vi "Dresden R2R Sputter 03.02.2018 IY24.vi"() -> ()   [LabVIEW 2009] (continued)
              }
              frame #1 {
                n8490 = call "Elapsed Time120"("Reset"=w13371) -> ("Elapsed Time (s)"=w13370:dbl)  [unwired: 11 in, 7 out]
                n8491 = Greater?(x=w13370, y=5.0) -> (0:w13368:bool)
              }
            }
            n8492 = local write "ch3_cc_fail_top"(w13330) -> ()
            n8493 = local write "Ch3_Ch_cc_fail"(w13330) -> ()
          }
        }
        n8494 = case shown="False" w13260 {
          frame #0 {
            n8495 = local read "Ch3_Trns_gv_bp2_do"() -> (w13266:bool)
            n8496 = local read "Ch3_Trns_gv_bp2_di"() -> (w13267:bool)
            n8497 = Exclusive Or(1:w13266, 2:w13267) -> (0:w13265:bool)
            n8498 = feedback #272() -> (w13264:bool)  [unwired: 1 in]
            n8499 = case shown="True" w13265 {
              tunnel: [TRUE FALSE] -> w13263
              tunnel: w13264 -> [_ w13273]
              tunnel: [FALSE w13270] -> w13262
              frame #0 {
              }
              frame #1 {
                n8500 = call "Elapsed Time156"("Reset"=w13273) -> ("Elapsed Time (s)"=w13272:dbl)  [unwired: 11 in, 7 out]
                n8501 = Greater?(x=w13272, y=5.0) -> (0:w13270:bool)
              }
            }
            n8502 = local write "Ch3_trns_gv_bp2_fail_front"(w13262) -> ()
            n8503 = local write "Ch3_Trns_gv_bp2_fail"(w13262) -> ()
            n8504 = local write "ch3_trns_gv_bp2_on_top"(w13262) -> ()
          }
          frame #1 {
            w13275 = TRUE ("Ch_bv_fail(ch3)L")
            n8505 = local write "Ch3_Trns_gv_bp2_fail"(w13275) -> ()
            n8506 = local write "Ch3_trns_gv_bp2_fail_front"(w13275) -> ()
            n8507 = local write "ch3_trns_gv_bp2_on_top"(w13275) -> ()
          }
        }
        n8508 = case shown="False" w13259 {
          frame #0 {
          }
          frame #1 {
          }
        }
        n8509 = case shown="False" w13261 {
          frame #0 {
            w13276 = TRUE ("Mp_fail(ch3)")
            n8510 = local write "Trns_gv_3_4_fail"(w13276) -> ()
            n8511 = local write "ch3_sov_Ar_fail_top"(w13276) -> ()
            n8512 = local write "gv top failed ch4_3"(w13276) -> ()
            n8513 = local write "gv front failed ch4_3"(w13276) -> ()
            n8514 = local write "gv top failed_ch3_4"(w13276) -> ()
            n8515 = local write "gv front failed_ch3_4"(w13276) -> ()
            n8516 = local write "Ch3_Trns_gv_bp_fail"(w13276) -> ()
            n8517 = local write "ch3_trns_gv_bp_on_top"(w13276) -> ()
            n8518 = local write "Ch3_trns_gv_bp_fail_front"(w13276) -> ()
            n8519 = local write "chamber 3 top piston failed"(w13276) -> ()
          }
          frame #1 {
            n8520 = local read "Ch3_Sov_Ar_do"() -> (w13296:bool)
            n8521 = local read "Ch3_Sov_Ar_di"() -> (w13297:bool)
            n8522 = Exclusive Or(1:w13296, 2:w13297) -> (0:w13298:bool)
            n8523 = feedback #273() -> (w13299:bool)  [unwired: 1 in]
            n8524 = case shown="True" w13298 {
              tunnel: [TRUE FALSE] -> w13300
              tunnel: w13299 -> [_ w13327]
              tunnel: [FALSE w13324] -> w13283
              frame #0 {
              }
              frame #1 {
                n8525 = call "Elapsed Time121"("Reset"=w13327) -> ("Elapsed Time (s)"=w13326:dbl)  [unwired: 11 in, 7 out]
                n8526 = Greater?(x=w13326, y=5.0) -> (0:w13324:bool)
              }
            }
            n8527 = local write "ch3_sov_Ar_fail_top"(w13283) -> ()
            n8528 = local read "Ch3_Trns_gv_open_di"() -> (w13294:bool)
            n8529 = local read "Ch3_Trns_gv_open_do"() -> (w13295:bool)
            n8530 = Exclusive Or(1:w13295, 2:w13294) -> (0:w13293:bool)
            n8531 = feedback #274() -> (w13292:bool)  [unwired: 1 in]
            n8532 = case shown="True" w13293 {
              tunnel: [TRUE FALSE] -> w13291
              tunnel: w13292 -> [_ w13320]
              tunnel: [FALSE w13317] -> w13290
              frame #0 {
              }
              frame #1 {
                n8533 = call "Elapsed Time139"("Reset"=w13320) -> ("Elapsed Time (s)"=w13319:dbl)  [unwired: 11 in, 7 out]
                n8534 = Greater?(x=w13319, y=60.0) -> (0:w13317:bool)
              }
            }
            n8535 = local write "gv top failed_ch3_4"(w13290) -> ()
            n8536 = local write "gv front failed_ch3_4"(w13290) -> ()
            n8537 = local write "Trns_gv_3_4_fail"(w13290) -> ()
            n8538 = local write "gv top failed ch4_3"(w13290) -> ()
            n8539 = local write "gv front failed ch4_3"(w13290) -> ()
            n8540 = local read "Ch3_Trns_gv_bp_do"() -> (w13285:bool)
            n8541 = local read "Ch3_Trns_gv_bp_di"() -> (w13286:bool)
            n8542 = Exclusive Or(1:w13285, 2:w13286) -> (0:w13287:bool)
            n8543 = feedback #275() -> (w13288:bool)  [unwired: 1 in]
            n8544 = case shown="True" w13287 {
              tunnel: [TRUE FALSE] -> w13289
              tunnel: w13288 -> [_ w13313]
              tunnel: [FALSE w13310] -> w13284
              frame #0 {
              }
              frame #1 {
                n8545 = call "Elapsed Time155"("Reset"=w13313) -> ("Elapsed Time (s)"=w13312:dbl)  [unwired: 11 in, 7 out]
                n8546 = Greater?(x=w13312, y=5.0) -> (0:w13310:bool)
              }
            }
            n8547 = local write "Ch3_Trns_gv_bp_fail"(w13284) -> ()
            n8548 = local write "Ch3_trns_gv_bp_fail_front"(w13284) -> ()
            n8549 = local write "ch3_trns_gv_bp_on_top"(w13284) -> ()
            n8550 = local read "Ch3_Cst_fix_down_di"() -> (w13279:bool)
            n8551 = local read "Ch3_Cst_fix_do"() -> (w13278:bool)
            n8552 = Exclusive Or(1:w13279, 2:w13278) -> (0:w13282:bool)
            n8553 = feedback #276() -> (w13280:bool)  [unwired: 1 in]
            n8554 = case shown="True" w13282 {
              tunnel: [TRUE FALSE] -> w13281
              tunnel: w13280 -> [_ w13306]
              tunnel: [FALSE w13303] -> w13277
              frame #0 {
              }
              frame #1 {
                n8555 = call "Elapsed Time188"("Reset"=w13306) -> ("Elapsed Time (s)"=w13305:dbl)  [unwired: 11 in, 7 out]
                n8556 = Greater?(x=w13305, y=60.0) -> (0:w13303:bool)
              }
            }
            n8557 = local write "chamber 3 top piston failed"(w13277) -> ()
          }
        }
      }
    }
  }
  n8558 = call <vilib>:"MB Serial Init.vi"(10:i32? 115200 ("Baud Rate"), 11:"Merobel Tension Controller 1") -> (0:w803, 3:w804)  [unwired: 8 in]
  n8559 = call <vilib>:"MB Serial Init.vi"("Timeout"=i32? 2000, "Mode"=w787, "Parity"=w785, "Baud Rate"=i32? 9600, "VISA resource name"="Moxa I/O Center") -> ("error out"=w747:errorcluster, "VISA resource name out"=w748:refnum<visa-resource-name>)  [unwired: 2 in, 3 out]
  n8560 = call <vilib>:"MB Serial Init.vi"("Timeout"=i32? 2000, "Mode"=w28, "Parity"=w30, "Baud Rate"=i32? 9600, "VISA resource name"="Autonics Counter") -> ("error out"=w26:errorcluster, "VISA resource name out"=w27:refnum<visa-resource-name>)  [unwired: 2 in, 3 out]
  n8561 = while {
    tunnel: w830 -> [w13411]
    tunnel: w829 -> [w13410]
    tunnel: [w13409] -> w808
    tunnel: [w13408] -> w807
    stop <- i16? 0 stop-if-true
    n8562 = Wait Until Next ms Multiple(millisecond multiple=i32? 300) -> ()  [unwired: 1 out]
    n8563 = stacked-sequence {
      tunnel: w13411 -> [w13416 _ _ _]
      tunnel: w13410 -> [w13415 _ _ _]
      tunnel: [_ _ _ w14644] -> w13409
      tunnel: [_ _ _ w14643] -> w13408
      frame #0 {
        n8564 = Or(x="Tp1_Set_speed", y="Tp1_auto_set_speed") -> (x .or. y?=w13434)
        n8565 = Compound Arithmetic op=OR("Tp1_Start", "Tp_start_ch1_gui", "Tp1_auto_start") -> (w13417)
        n8566 = Compound Arithmetic op=OR("Tp1_Stop", "Tp_stop_ch1_gui", "Tp1_auto_stop") -> (w13419)
        n8567 = Or(x="Tp1_Low_speed", y="Tp1_auto_low_speed") -> (x .or. y?=w13432)
        n8568 = Or(x="Tp1_Normal_speed", y="Tp1_auto_normal_speed") -> (x .or. y?=w13428)
        n8569 = case shown="True" w13417 {
          tunnel: [i16? 0 w13443] -> w13414
          frame #0 {
          }
          frame #1 {
            n8570 = local read "Ch1_Tp_start_safety"() -> (w13444)
            n8571 = case shown="False" w13444 {
              tunnel: [i16? 0 T/1] -> w13443
              frame #0 {
                n8572 = local write "Tp1_auto_start"(i16? 0 ("Tp1_auto_start")) -> ()
                n8573 = local write "Error Message"("TP can not be started.\nReason:\n*MP can not be open. \n *TP-BV can not be  open.\n *Pressure difference between\n       chamber and pipeline \nnot suitable.\n" ("Error Message")) -> ()
              }
              frame #1 {
              }
            }
          }
        }
        n8574 = Build Array(i16? 0, w13414, w13419, w13434, w13432, w13428, "Tp1_Start_initial", "Tp1_Stop_initial") -> (w13440)
        n8575 = Boolean Array To Number(Boolean array=w13440) -> (number=w13441)
        n8576 = Mantissa & Exponent(0:w13441) -> (2:w13439)  [unwired: 1 out]
        n8577 = case shown="0, Default" w13439 {
          tunnel: w13416 -> [w13452 w13564 w13600 w13641 w13683 w13717 w13751 w13785]
          tunnel: w13415 -> [w13451 w13563 w13599 w13640 w13682 w13716 w13750 w13784]
          tunnel: [w13450 w13562 w13598 w13639 w13681 w13715 w13749 w13783] -> w13438
          tunnel: [w13449 w13561 w13597 w13638 w13680 w13714 w13748 w13782] -> w13418
          frame #0 {
            n8578 = stacked-sequence {
              tunnel: w13452 -> [w13468 _]
              tunnel: w13451 -> [w13467 _]
              tunnel: [_ w13519] -> w13450
              tunnel: [_ w13518] -> w13449
              frame #0 {
                # "Address"
                # "Address"
                n8579 = Concatenate Strings("001" ("write buffer"), "00" ("string"), "309" ("string"), "02" ("string"), "=?" ("string")) -> (w13477)
                n8580 = String To Byte Array(string=w13477) -> (unsigned byte array=w13482)
                n8581 = for {
                  tunnel: w13482 -> [w13514] mode=indexing
                  shift-right: [w13512] -> w13484
                  shift-left: i16? 0 -> [w13513]
                  n8582 = Add(x=w13514, y=w13513) -> (x+y=w13512)
                }
                n8583 = Number To Decimal String(number=w13484) -> (decimal integer string=w13479)  [unwired: 1 in]
                n8584 = String Length(string=w13479) -> (length=w13480)
                n8585 = case shown="3" w13480 {
                  tunnel: w13479 -> [_ w13507 w13510 w13511]
                  tunnel: [data[5B] w13505 w13508 w13511] -> w13478
                  frame #0 {
                  }
                  frame #1 {
                    n8586 = Concatenate Strings("00" ("string"), w13507) -> (w13505)
                  }
                  frame #2 {
                    n8587 = Concatenate Strings("0" ("string"), w13510) -> (w13508)
                  }
                  frame #3 {
                  }
                }
                n8588 = Concatenate Strings(w13477, w13478, "\n") -> (w13469)
                n8589 = VISA Write(VISA resource name=w13468, write buffer=w13469, error in (no error)=w13467) -> (VISA resource name out=w13472, error out=w13471)  [unwired: 1 out]
                n8590 = stacked-sequence {
                  tunnel: [w13503] -> w13474
                  tunnel: w13472 -> [w13503]
                  tunnel: [w13502] -> w13473
                  tunnel: w13471 -> [w13502]
                  frame #0 {
                    n8591 = Wait (ms)(milliseconds to wait=i32? 100) -> ()  [unwired: 1 out]
                  }
                }
                n8592 = property class="Instr"(reference=w13474, error in=w13473) -> (reference out=w13476, error out=w13475, "Serial Settings:Number of Bytes at Serial Port"=w13470)
                n8593 = VISA Read(VISA resource name=w13476, byte count=w13470, error in (no error)=w13475) -> (VISA resource name out=w13459, read buffer=w13453, error out=w13458)  [unwired: 1 out]
                "Read_data" <- w13453
                n8594 = String Length(string=w13453) -> (length=w13466)
                n8595 = Not Equal To 0?(x=w13466) -> (x != 0?=w13457)
                n8596 = feedback #277() -> (w13455)  [unwired: 1 in]
                n8597 = Concatenate Strings("001" ("regular expression"), "1030906" ("regular expression")) -> (w13465)
                n8598 = case shown="False" w13457 {
                  tunnel: [w13492 T/1] -> w13454
                  tunnel: [i16? 0 T/1] -> w13456
                  tunnel: w13455 -> [w13490 _]
                  frame #0 {
                    n8599 = call "Elapsed Time131"(2:w13490) -> (16:w13493)  [unwired: 11 in, 7 out]
                    n8600 = Greater?(x=w13493, y=dbl? 5.0) -> (0:w13492)
                  }
                  frame #1 {
                  }
                }
                "Com_ok" <- w13454
                n8601 = Match Pattern(string=w13453, regular expression=w13465) -> (after substring=w13460)  [unwired: 4 out]
                n8602 = String Length(string=w13460) -> (length=w13462)
                n8603 = Not Equal To 0?(x=w13462) -> (x != 0?=w13461)
                n8604 = case shown="True" w13461 {
                  tunnel: w13460 -> [_ w13498]
                  frame #0 {
                  }
                  frame #1 {
                    n8605 = String Subset(string=w13498, length (rest)=i32? 6 ("length (rest)")) -> (substring=w13499)  [unwired: 1 out]
                    n8606 = Decimal String To Number(string=w13499) -> (number=→"Tp1_speed_gui" →"Turbo_pump_speed 7")  [unwired: 3 out]
                  }
                }
              }
              frame #1 {
                # "Address"
                # "Address"
                n8607 = Concatenate Strings("001" ("write buffer"), "00" ("string"), "307" ("string"), "02" ("string"), "=?" ("string")) -> (w13532)
                n8608 = String To Byte Array(string=w13532) -> (unsigned byte array=w13537)
                n8609 = for {
                  tunnel: w13537 -> [w13558] mode=indexing
                  shift-right: [w13556] -> w13539
                  shift-left: i16? 0 -> [w13557]
                  n8610 = Add(x=w13558, y=w13557) -> (x+y=w13556)
                }
                n8611 = Number To Decimal String(number=w13539) -> (decimal integer string=w13534)  [unwired: 1 in]
                n8612 = String Length(string=w13534) -> (length=w13535)
                n8613 = case shown="0, Default" w13535 {
                  tunnel: w13534 -> [_ w13551 w13554 w13555]
                  tunnel: [data[5B] w13549 w13552 w13555] -> w13533
                  frame #0 {
                  }
                  frame #1 {
                    n8614 = Concatenate Strings("00" ("string"), w13551) -> (w13549)
                  }
                  frame #2 {
                    n8615 = Concatenate Strings("0" ("string"), w13554) -> (w13552)
                  }
                  frame #3 {
                  }
                }
                n8616 = Concatenate Strings(w13532, w13533, "\n") -> (w13524)
                n8617 = VISA Write(VISA resource name=w13517, write buffer=w13524, error in (no error)=w13515) -> (VISA resource name out=w13527, error out=w13526)  [unwired: 1 out]
                n8618 = stacked-sequence {
                  tunnel: [w13547] -> w13529
                  tunnel: w13527 -> [w13547]
                  tunnel: [w13546] -> w13528
                  tunnel: w13526 -> [w13546]
                  frame #0 {
                    n8619 = Wait (ms)(milliseconds to wait=i32? 100) -> ()  [unwired: 1 out]
                  }
                }
                n8620 = property class="Instr"(reference=w13529, error in=w13528) -> (reference out=w13531, error out=w13530, "Serial Settings:Number of Bytes at Serial Port"=w13525)
                n8621 = VISA Read(VISA resource name=w13531, byte count=w13525, error in (no error)=w13530) -> (VISA resource name out=w13519, read buffer=w13523, error out=w13518)  [unwired: 1 out]
                "Read_data 3" <- w13523
                n8622 = Concatenate Strings("001" ("regular expression"), "1030706" ("regular expression")) -> (w13522)
                n8623 = Match Pattern(string=w13523, regular expression=w13522) -> (after substring=→"after substring")  [unwired: 4 out]
              }
            }
          }
          frame #1 {
            # "Cheksum 3 haneli olmalı"
            # "Address"
            n8624 = Concatenate Strings("001" ("write buffer"), "10" ("string"), "010" ("string"), "06" ("string"), "111111" ("string")) -> (w13568)
            n8625 = String To Byte Array(string=w13568) -> (unsigned byte array=w13573)
            n8626 = for {
              tunnel: w13573 -> [w13594] mode=indexing
              shift-right: [w13592] -> w13575
              shift-left: i16? 0 -> [w13593]
              n8627 = Add(x=w13594, y=w13593) -> (x+y=w13592)
            }
            n8628 = Number To Decimal String(number=w13575) -> (decimal integer string=w13570)  [unwired: 1 in]
            "decimal integer string" <- w13570
            n8629 = String Length(string=w13570) -> (length=w13571)
            n8630 = local write "Tp1_auto_start"(i16? 0 ("Tp1_auto_start")) -> ()
            n8631 = case shown="1" w13571 {
              tunnel: w13570 -> [_ w13587 w13590 w13591]
              tunnel: [data[5B] w13585 w13588 w13591] -> w13569
              frame #0 {
              }
              frame #1 {
                n8632 = Concatenate Strings("00" ("string"), w13587) -> (w13585)
              }
              frame #2 {
                n8633 = Concatenate Strings("0" ("string"), w13590) -> (w13588)
              }
              frame #3 {
              }
            }
            n8634 = local write "Tp1_stop_cmnd"(i16? 0 ("Tp1_stop_cmnd")) -> ()
            n8635 = Concatenate Strings(w13568, w13569, "\n") -> (w13565)
            n8636 = VISA Write(VISA resource name=w13564, write buffer=w13565, error in (no error)=w13563) -> (VISA resource name out=w13567, error out=w13566)  [unwired: 1 out]
            n8637 = stacked-sequence {
              tunnel: [w13583] -> w13562
              tunnel: w13567 -> [w13583]
              tunnel: [w13582] -> w13561
              tunnel: w13566 -> [w13582]
              frame #0 {
                n8638 = Wait (ms)(milliseconds to wait=i32? 100) -> ()  [unwired: 1 out]
              }
            }
          }
          frame #2 {
            # "Cheksum 3 haneli olmalı"
            # "Address"
            n8639 = Concatenate Strings("001" ("write buffer"), "10" ("string"), "010" ("string"), "06" ("string"), "000000" ("string")) -> (w13604)
            n8640 = String To Byte Array(string=w13604) -> (unsigned byte array=w13609)
            n8641 = for {
              tunnel: w13609 -> [w13630] mode=indexing
              shift-right: [w13628] -> w13611
              shift-left: i16? 0 -> [w13629]
              n8642 = Add(x=w13630, y=w13629) -> (x+y=w13628)
            }
            n8643 = Number To Decimal String(number=w13611) -> (decimal integer string=w13606)  [unwired: 1 in]
            n8644 = local write "Tp1_auto_stop"(i16? 0 ("Tp1_auto_stop")) -> ()
            n8645 = String Length(string=w13606) -> (length=w13607)
            n8646 = case shown="0, Default" w13607 {
              tunnel: w13606 -> [_ w13623 w13626 w13627]
              tunnel: [data[5B] w13621 w13624 w13627] -> w13605
              frame #0 {
              }
              frame #1 {
                n8647 = Concatenate Strings("00" ("string"), w13623) -> (w13621)
              }
              frame #2 {
                n8648 = Concatenate Strings("0" ("string"), w13626) -> (w13624)
              }
              frame #3 {
              }
            }
            n8649 = Concatenate Strings(w13604, w13605, "\n") -> (w13601)
            n8650 = VISA Write(VISA resource name=w13600, write buffer=w13601, error in (no error)=w13599) -> (VISA resource name out=w13603, error out=w13602)  [unwired: 1 out]
            n8651 = stacked-sequence {
              tunnel: [w13619] -> w13598
              tunnel: w13603 -> [w13619]
              tunnel: [w13618] -> w13597
              tunnel: w13602 -> [w13618]
              frame #0 {
                n8652 = Wait (ms)(milliseconds to wait=i32? 100) -> ()  [unwired: 1 out]
              }
            }
            "Tp1_stop_cmnd" <- T/1 ("Tp_stop_cmnd")
          }
          frame #3 {
            # "Cheksum 3 haneli olmalı"
            # "Address"
            n8653 = Multiply(x="Low_speed_value", y=data[16B]) -> (x*y=w13635)
            n8654 = To Unsigned Long Integer(number=w13635) -> (unsigned 32bit integer=w13634)
            n8655 = Number To Decimal String(number=w13634) -> (decimal integer string=w13632)  [unwired: 1 out]
            n8656 = String Length(string=w13632) -> (length=w13633)
            n8657 = case shown="0, Default" w13633 {
              tunnel: w13632 -> [_ w13661 w13664 w13665]
              tunnel: [data[5B] w13660 w13663 w13665] -> w13631
              frame #0 {
              }
              frame #1 {
                n8658 = Concatenate Strings(w13661, "00" ("string")) -> (w13660)
              }
              frame #2 {
                n8659 = Concatenate Strings(w13664, "0" ("string")) -> (w13663)
              }
              frame #3 {
              }
            }
            n8660 = Concatenate Strings("001" ("write buffer"), "10" ("string"), "707" ("string"), "06" ("string"), "00" ("string"), w13631) -> (w13645)
            n8661 = String To Byte Array(string=w13645) -> (unsigned byte array=w13650)
            n8662 = for {
              tunnel: w13650 -> [w13679] mode=indexing
              shift-right: [w13677] -> w13652
              shift-left: i16? 0 -> [w13678]
              n8663 = Add(x=w13679, y=w13678) -> (x+y=w13677)
            }
            n8664 = Number To Decimal String(number=w13652) -> (decimal integer string=w13647)  [unwired: 1 in]
            n8665 = String Length(string=w13647) -> (length=w13648)
            n8666 = case shown="3" w13648 {
              tunnel: w13647 -> [_ w13672 w13675 w13676]
              tunnel: [data[5B] w13670 w13673 w13676] -> w13646
              frame #0 {
              }
              frame #1 {
                n8667 = Concatenate Strings("00" ("string"), w13672) -> (w13670)
              }
              frame #2 {
                n8668 = Concatenate Strings("0" ("string"), w13675) -> (w13673)
              }
              frame #3 {
              }
            }
            n8669 = Concatenate Strings(w13645, w13646, "\n") -> (w13642)
            n8670 = VISA Write(VISA resource name=w13641, write buffer=w13642, error in (no error)=w13640) -> (VISA resource name out=w13644, error out=w13643)  [unwired: 1 out]
            n8671 = stacked-sequence {
              tunnel: [w13668] -> w13639
              tunnel: w13644 -> [w13668]
              tunnel: [w13667] -> w13638
              tunnel: w13643 -> [w13667]
              frame #0 {
                n8672 = Wait (ms)(milliseconds to wait=i32? 100) -> ()  [unwired: 1 out]
              }
            }
          }
          frame #4 {
            # "Cheksum 3 haneli olmalı"
            # "Address"
            n8673 = Concatenate Strings("001" ("write buffer"), "10" ("string"), "026" ("string"), "03" ("string"), "001" ("string")) -> (w13687)
            n8674 = String To Byte Array(string=w13687) -> (unsigned byte array=w13692)
            n8675 = for {
              tunnel: w13692 -> [w13713] mode=indexing
              shift-right: [w13711] -> w13694
              shift-left: i16? 0 -> [w13712]
              n8676 = Add(x=w13713, y=w13712) -> (x+y=w13711)
            }
            n8677 = Number To Decimal String(number=w13694) -> (decimal integer string=w13689)  [unwired: 1 in]
            n8678 = String Length(string=w13689) -> (length=w13690)
            n8679 = case shown="0, Default" w13690 {
              tunnel: w13689 -> [_ w13706 w13709 w13710]
              tunnel: [data[5B] w13704 w13707 w13710] -> w13688
              frame #0 {
              }
              frame #1 {
                n8680 = Concatenate Strings("00" ("string"), w13706) -> (w13704)
              }
              frame #2 {
                n8681 = Concatenate Strings("0" ("string"), w13709) -> (w13707)
              }
              frame #3 {
              }
            }
            n8682 = Concatenate Strings(w13687, w13688, "\n") -> (w13684)
            n8683 = VISA Write(VISA resource name=w13683, write buffer=w13684, error in (no error)=w13682) -> (VISA resource name out=w13686, error out=w13685)  [unwired: 1 out]
            n8684 = stacked-sequence {
              tunnel: [w13702] -> w13681
              tunnel: w13686 -> [w13702]
              tunnel: [w13701] -> w13680
              tunnel: w13685 -> [w13701]
              frame #0 {
                n8685 = Wait (ms)(milliseconds to wait=i32? 100) -> ()  [unwired: 1 out]
              }
            }
          }
          frame #5 {
            # "Cheksum 3 haneli olmalı"
            # "Address"
            n8686 = Concatenate Strings("001" ("write buffer"), "10" ("string"), "026" ("string"), "03" ("string"), "000" ("string")) -> (w13721)
            n8687 = String To Byte Array(string=w13721) -> (unsigned byte array=w13726)
            n8688 = for {
              tunnel: w13726 -> [w13747] mode=indexing
              shift-right: [w13745] -> w13728
              shift-left: i16? 0 -> [w13746]
              n8689 = Add(x=w13747, y=w13746) -> (x+y=w13745)
            }
            n8690 = Number To Decimal String(number=w13728) -> (decimal integer string=w13723)  [unwired: 1 in]
            n8691 = String Length(string=w13723) -> (length=w13724)
            n8692 = case shown="0, Default" w13724 {
              tunnel: w13723 -> [_ w13740 w13743 w13744]
              tunnel: [data[5B] w13738 w13741 w13744] -> w13722
              frame #0 {
              }
              frame #1 {
                n8693 = Concatenate Strings("00" ("string"), w13740) -> (w13738)
              }
              frame #2 {
                n8694 = Concatenate Strings("0" ("string"), w13743) -> (w13741)
              }
              frame #3 {
              }
            }
            n8695 = Concatenate Strings(w13721, w13722, "\n") -> (w13718)
            n8696 = VISA Write(VISA resource name=w13717, write buffer=w13718, error in (no error)=w13716) -> (VISA resource name out=w13720, error out=w13719)  [unwired: 1 out]
            n8697 = stacked-sequence {
              tunnel: [w13736] -> w13715
              tunnel: w13720 -> [w13736]
              tunnel: [w13735] -> w13714
              tunnel: w13719 -> [w13735]
              frame #0 {
                n8698 = Wait (ms)(milliseconds to wait=i32? 100) -> ()  [unwired: 1 out]
              }
            }
          }
          frame #6 {
            # "Cheksum 3 haneli olmalı"
            # "Address"
            n8699 = Concatenate Strings("001" ("write buffer"), "10" ("string"), "023" ("string"), "06" ("string"), "111111" ("string")) -> (w13755)
            n8700 = String To Byte Array(string=w13755) -> (unsigned byte array=w13760)
            n8701 = for {
              tunnel: w13760 -> [w13781] mode=indexing
              shift-right: [w13779] -> w13762
              shift-left: i16? 0 -> [w13780]
              n8702 = Add(x=w13781, y=w13780) -> (x+y=w13779)
            }
            n8703 = Number To Decimal String(number=w13762) -> (decimal integer string=w13757)  [unwired: 1 in]
            n8704 = String Length(string=w13757) -> (length=w13758)
            n8705 = case shown="0, Default" w13758 {
              tunnel: w13757 -> [_ w13774 w13777 w13778]
              tunnel: [data[5B] w13772 w13775 w13778] -> w13756
              frame #0 {
              }
              frame #1 {
                n8706 = Concatenate Strings("00" ("string"), w13774) -> (w13772)
              }
              frame #2 {
                n8707 = Concatenate Strings("0" ("string"), w13777) -> (w13775)
              }
              frame #3 {
              }
            }
            n8708 = Concatenate Strings(w13755, w13756, "\n") -> (w13752)
            n8709 = VISA Write(VISA resource name=w13751, write buffer=w13752, error in (no error)=w13750) -> (VISA resource name out=w13754, error out=w13753)  [unwired: 1 out]
            n8710 = stacked-sequence {
              tunnel: [w13770] -> w13749
              tunnel: w13754 -> [w13770]
              tunnel: [w13769] -> w13748
              tunnel: w13753 -> [w13769]
              frame #0 {
                n8711 = Wait (ms)(milliseconds to wait=i32? 100) -> ()  [unwired: 1 out]
              }
            }
          }
          frame #7 {
            # "Cheksum 3 haneli olmalı"
            # "Address"
            n8712 = Concatenate Strings("001" ("write buffer"), "10" ("string"), "023" ("string"), "06" ("string"), "000000" ("string")) -> (w13789)
            n8713 = String To Byte Array(string=w13789) -> (unsigned byte array=w13794)
            n8714 = for {
              tunnel: w13794 -> [w13815] mode=indexing
              shift-right: [w13813] -> w13796
              shift-left: i16? 0 -> [w13814]
              n8715 = Add(x=w13815, y=w13814) -> (x+y=w13813)
            }
            n8716 = Number To Decimal String(number=w13796) -> (decimal integer string=w13791)  [unwired: 1 in]
            n8717 = String Length(string=w13791) -> (length=w13792)
            n8718 = case shown="0, Default" w13792 {
              tunnel: w13791 -> [_ w13808 w13811 w13812]
              tunnel: [data[5B] w13806 w13809 w13812] -> w13790
              frame #0 {
              }
              frame #1 {
                n8719 = Concatenate Strings("00" ("string"), w13808) -> (w13806)
              }
              frame #2 {
                n8720 = Concatenate Strings("0" ("string"), w13811) -> (w13809)
              }
              frame #3 {
              }
            }
            n8721 = Concatenate Strings(w13789, w13790, "\n") -> (w13786)
            n8722 = VISA Write(VISA resource name=w13785, write buffer=w13786, error in (no error)=w13784) -> (VISA resource name out=w13788, error out=w13787)  [unwired: 1 out]
            n8723 = stacked-sequence {
              tunnel: [w13804] -> w13783
              tunnel: w13788 -> [w13804]
              tunnel: [w13803] -> w13782
              tunnel: w13787 -> [w13803]
              frame #0 {
                n8724 = Wait (ms)(milliseconds to wait=i32? 100) -> ()  [unwired: 1 out]
              }
            }
          }
        }
      }
      frame #1 {
        n8725 = Compound Arithmetic op=OR("Tp2_start", "Tp_start_ch2_gui", "Tp2_auto_start") -> (w13820)
        n8726 = Or(x="Tp2_low_speed", y="Tp2_auto_low_speed") -> (x .or. y?=w13835)
        n8727 = Or(x="Tp2_normal_speed", y="Tp2_auto_normal_speed") -> (x .or. y?=w13830)
        n8728 = Compound Arithmetic op=OR("Tp2_stop", "Tp_stop_ch2_gui", "Tp2_auto_stop") -> (w13822)
        n8729 = Or(x="Tp2_set_speed", y="Tp2_auto_set_speed") -> (x .or. y?=w13836)
        n8730 = case shown="True" w13820 {
          tunnel: [i16? 0 w13845] -> w13819
          frame #0 {
          }
          frame #1 {
            n8731 = local read "Ch2_Tp_start_safety"() -> (w13846)
            n8732 = case shown="False" w13846 {
              tunnel: [i16? 0 T/1] -> w13845
              frame #0 {
                n8733 = local write "Tp2_auto_start"(i16? 0 ("Tp1_auto_start")) -> ()
                n8734 = local write "Error Message"("TP can not be started.\nReason:\n*MP can not be open. \n    *TP-BV can not be open.\n *Pressure difference between\nchamber and pipeline \nnot suitable.\n" ("Error Message")) -> ()
              }
              frame #1 {
              }
            }
          }
        }
        n8735 = Build Array(i16? 0, w13819, w13822, w13836, w13835, w13830, "Tp2_start_initial", "Tp2_stop_initial") -> (w13842)
        n8736 = Boolean Array To Number(Boolean array=w13842) -> (number=w13843)
        n8737 = Mantissa & Exponent(0:w13843) -> (2:w13840)  [unwired: 1 out]
        n8738 = case shown="0, Default" w13840 {
          tunnel: w13839 -> [w13851 w13966 w14002 w14043 w14085 w14119 w14153 w14187]
          tunnel: w13821 -> [w13852 w13965 w14001 w14042 w14084 w14118 w14152 w14186]
          tunnel: [w13854 w13964 w14000 w14041 w14083 w14117 w14151 w14185] -> w13817
          tunnel: [w13853 w13963 w13999 w14040 w14082 w14116 w14150 w14184] -> w13816
          frame #0 {
            n8739 = stacked-sequence {
              tunnel: w13851 -> [w13870 _]
              tunnel: w13852 -> [w13869 _]
              tunnel: [_ w13921] -> w13854
              tunnel: [_ w13920] -> w13853
              frame #0 {
                # "Address"
                # "Cheksum 3 haneli olmalı"
                # "Address"
                n8740 = Concatenate Strings("002" ("write buffer"), "00" ("string"), "309" ("string"), "02" ("string"), "=?" ("string")) -> (w13879)
                n8741 = String To Byte Array(string=w13879) -> (unsigned byte array=w13884)
                n8742 = for {
                  tunnel: w13884 -> [w13916] mode=indexing
                  shift-right: [w13914] -> w13886
                  shift-left: i16? 0 -> [w13915]
                  n8743 = Add(x=w13916, y=w13915) -> (x+y=w13914)
                }
                n8744 = Number To Decimal String(number=w13886) -> (decimal integer string=w13881)  [unwired: 1 in]
                n8745 = String Length(string=w13881) -> (length=w13882)
                n8746 = case shown="0, Default" w13882 {
                  tunnel: w13881 -> [_ w13909 w13912 w13913]
                  tunnel: [data[5B] w13907 w13910 w13913] -> w13880
                  frame #0 {
                  }
                  frame #1 {
                    n8747 = Concatenate Strings("00" ("string"), w13909) -> (w13907)
                  }
                  frame #2 {
                    n8748 = Concatenate Strings("0" ("string"), w13912) -> (w13910)
                  }
                  frame #3 {
                  }
                }
                n8749 = Concatenate Strings(w13879, w13880, "\n") -> (w13871)
                n8750 = VISA Write(VISA resource name=w13870, write buffer=w13871, error in (no error)=w13869) -> (VISA resource name out=w13874, error out=w13873)  [unwired: 1 out]
                n8751 = stacked-sequence {
                  tunnel: [w13905] -> w13876
                  tunnel: w13874 -> [w13905]
                  tunnel: [w13904] -> w13875
                  tunnel: w13873 -> [w13904]
                  frame #0 {
                    n8752 = Wait (ms)(milliseconds to wait=i32? 100) -> ()  [unwired: 1 out]
                  }
                }
                n8753 = property class="Instr"(reference=w13876, error in=w13875) -> (reference out=w13878, error out=w13877, "Serial Settings:Number of Bytes at Serial Port"=w13872)
                n8754 = VISA Read(VISA resource name=w13878, byte count=w13872, error in (no error)=w13877) -> (VISA resource name out=w13860, read buffer=w13867, error out=w13859)  [unwired: 1 out]
                "Read_data 4" <- w13867
                n8755 = String Length(string=w13867) -> (length=w13868)
                n8756 = Not Equal To 0?(x=w13868) -> (x != 0?=w13856)
                n8757 = Concatenate Strings("002" ("regular expression"), "1030906" ("regular expression")) -> (w13866)
                n8758 = Match Pattern(string=w13867, regular expression=w13866) -> (after substring=w13861)  [unwired: 4 out]
                n8759 = feedback #278() -> (w13857)  [unwired: 1 in]
                n8760 = String Length(string=w13861) -> (length=w13863)
                n8761 = Not Equal To 0?(x=w13863) -> (x != 0?=w13862)
                n8762 = case shown="True" w13856 {
                  tunnel: [i16? 0 w13896] -> w13855
                  tunnel: [T/1 i16? 0] -> w13858
                  tunnel: w13857 -> [_ w13894]
                  frame #0 {
                  }
                  frame #1 {
                    n8763 = call "Elapsed Time132"(2:w13894) -> (16:w13897)  [unwired: 11 in, 7 out]
                    n8764 = Greater?(x=w13897, y=dbl? 5.0) -> (0:w13896)
                  }
                }
                "Com_ok 2" <- w13855
                n8765 = case shown="True" w13862 {
                  tunnel: w13861 -> [_ w13900]
                  frame #0 {
                  }
                  frame #1 {
                    n8766 = String Subset(string=w13900, length (rest)=i32? 6 ("length (rest)")) -> (substring=w13901)  [unwired: 1 out]
                    n8767 = Decimal String To Number(string=w13901) -> (number=→"Tp2_speed_gui" →"Turbo_pump_speed 6")  [unwired: 3 out]
                  }
                }
              }
              frame #1 {
                # "Address"
                # "Cheksum 3 haneli olmalı"
                # "Address"
                n8768 = Concatenate Strings("002" ("write buffer"), "00" ("string"), "307" ("string"), "02" ("string"), "=?" ("string")) -> (w13934)
                n8769 = String To Byte Array(string=w13934) -> (unsigned byte array=w13939)
                n8770 = for {
                  tunnel: w13939 -> [w13960] mode=indexing
                  shift-right: [w13958] -> w13941
                  shift-left: i16? 0 -> [w13959]
                  n8771 = Add(x=w13960, y=w13959) -> (x+y=w13958)
                }
                n8772 = Number To Decimal String(number=w13941) -> (decimal integer string=w13936)  [unwired: 1 in]
                n8773 = String Length(string=w13936) -> (length=w13937)
                n8774 = case shown="0, Default" w13937 {
                  tunnel: w13936 -> [_ w13953 w13956 w13957]
                  tunnel: [data[5B] w13951 w13954 w13957] -> w13935
                  frame #0 {
                  }
                  frame #1 {
                    n8775 = Concatenate Strings("00" ("string"), w13953) -> (w13951)
                  }
                  frame #2 {
                    n8776 = Concatenate Strings("0" ("string"), w13956) -> (w13954)
                  }
                  frame #3 {
                  }
                }
                n8777 = Concatenate Strings(w13934, w13935, "\n") -> (w13926)
                n8778 = VISA Write(VISA resource name=w13918, write buffer=w13926, error in (no error)=w13919) -> (VISA resource name out=w13929, error out=w13928)  [unwired: 1 out]
                n8779 = stacked-sequence {
                  tunnel: [w13949] -> w13931
                  tunnel: w13929 -> [w13949]
                  tunnel: [w13948] -> w13930
                  tunnel: w13928 -> [w13948]
                  frame #0 {
                    n8780 = Wait (ms)(milliseconds to wait=i32? 100) -> ()  [unwired: 1 out]
                  }
                }
                n8781 = property class="Instr"(reference=w13931, error in=w13930) -> (reference out=w13933, error out=w13932, "Serial Settings:Number of Bytes at Serial Port"=w13927)
                n8782 = VISA Read(VISA resource name=w13933, byte count=w13927, error in (no error)=w13932) -> (VISA resource name out=w13921, read buffer=w13925, error out=w13920)  [unwired: 1 out]
                "Read_data 5" <- w13925
                n8783 = Concatenate Strings("002" ("regular expression"), "1030706" ("regular expression")) -> (w13924)
                n8784 = Match Pattern(string=w13925, regular expression=w13924) -> (after substring=→"after substring 2")  [unwired: 4 out]
              }
            }
          }
          frame #1 {
            # "Cheksum 3 haneli olmalı"
            # "Address"
            n8785 = Concatenate Strings("002" ("write buffer"), "10" ("string"), "010" ("string"), "06" ("string"), "111111" ("string")) -> (w13970)
            n8786 = String To Byte Array(string=w13970) -> (unsigned byte array=w13975)
            n8787 = for {
              tunnel: w13975 -> [w13996] mode=indexing
              shift-right: [w13994] -> w13977
              shift-left: i16? 0 -> [w13995]
              n8788 = Add(x=w13996, y=w13995) -> (x+y=w13994)
            }
            n8789 = Number To Decimal String(number=w13977) -> (decimal integer string=w13972)  [unwired: 1 in]
            n8790 = local write "Tp2_auto_start"(i16? 0 ("Tp2_auto_start")) -> ()
            n8791 = String Length(string=w13972) -> (length=w13973)
            n8792 = case shown="0, Default" w13973 {
              tunnel: w13972 -> [_ w13989 w13992 w13993]
              tunnel: [data[5B] w13987 w13990 w13993] -> w13971
              frame #0 {
              }
              frame #1 {
                n8793 = Concatenate Strings("00" ("string"), w13989) -> (w13987)
              }
              frame #2 {
                n8794 = Concatenate Strings("0" ("string"), w13992) -> (w13990)
              }
              frame #3 {
              }
            }
            n8795 = Concatenate Strings(w13970, w13971, "\n") -> (w13967)
            n8796 = local write "Tp2_stop_cmnd"(i16? 0 ("Tp2_stop_cmnd")) -> ()
            n8797 = VISA Write(VISA resource name=w13966, write buffer=w13967, error in (no error)=w13965) -> (VISA resource name out=w13969, error out=w13968)  [unwired: 1 out]
            n8798 = stacked-sequence {
              tunnel: [w13985] -> w13964
              tunnel: w13969 -> [w13985]
              tunnel: [w13984] -> w13963
              tunnel: w13968 -> [w13984]
              frame #0 {
                n8799 = Wait (ms)(milliseconds to wait=i32? 100) -> ()  [unwired: 1 out]
              }
            }
          }
          frame #2 {
            # "Cheksum 3 haneli olmalı"
            # "Address"
            n8800 = Concatenate Strings("002" ("write buffer"), "10" ("string"), "010" ("string"), "06" ("string"), "000000" ("string")) -> (w14006)
            n8801 = String To Byte Array(string=w14006) -> (unsigned byte array=w14011)
            n8802 = for {
              tunnel: w14011 -> [w14032] mode=indexing
              shift-right: [w14030] -> w14013
              shift-left: i16? 0 -> [w14031]
              n8803 = Add(x=w14032, y=w14031) -> (x+y=w14030)
            }
            n8804 = local write "Tp2_auto_stop"(i16? 0 ("Tp2_auto_stop")) -> ()
            n8805 = Number To Decimal String(number=w14013) -> (decimal integer string=w14008)  [unwired: 1 in]
            n8806 = String Length(string=w14008) -> (length=w14009)
            n8807 = case shown="0, Default" w14009 {
              tunnel: w14008 -> [_ w14025 w14028 w14029]
              tunnel: [data[5B] w14023 w14026 w14029] -> w14007
              frame #0 {
              }
              frame #1 {
                n8808 = Concatenate Strings("00" ("string"), w14025) -> (w14023)
              }
              frame #2 {
                n8809 = Concatenate Strings("0" ("string"), w14028) -> (w14026)
              }
              frame #3 {
              }
            }
            n8810 = Concatenate Strings(w14006, w14007, "\n") -> (w14003)
            n8811 = VISA Write(VISA resource name=w14002, write buffer=w14003, error in (no error)=w14001) -> (VISA resource name out=w14005, error out=w14004)  [unwired: 1 out]
            n8812 = stacked-sequence {
              tunnel: [w14021] -> w14000
              tunnel: w14005 -> [w14021]
              tunnel: [w14020] -> w13999
              tunnel: w14004 -> [w14020]
              frame #0 {
                n8813 = Wait (ms)(milliseconds to wait=i32? 100) -> ()  [unwired: 1 out]
              }
            }
            "Tp2_stop_cmnd" <- T/1 ("Tp2_stop_cmnd")
          }
          frame #3 {
            # "Cheksum 3 haneli olmalı"
            # "Address"
            n8814 = Multiply(x="Low_speed_value 2", y=data[16B]) -> (x*y=w14037)
            n8815 = To Unsigned Long Integer(number=w14037) -> (unsigned 32bit integer=w14036)
            n8816 = Number To Decimal String(number=w14036) -> (decimal integer string=w14034)  [unwired: 1 out]
            n8817 = String Length(string=w14034) -> (length=w14035)
            n8818 = case shown="3" w14035 {
              tunnel: w14034 -> [_ w14063 w14066 w14067]
              tunnel: [data[5B] w14062 w14065 w14067] -> w14033
              frame #0 {
              }
              frame #1 {
                n8819 = Concatenate Strings(w14063, "00" ("string")) -> (w14062)
              }
              frame #2 {
                n8820 = Concatenate Strings(w14066, "0" ("string")) -> (w14065)
              }
              frame #3 {
              }
            }
            n8821 = Concatenate Strings("002" ("write buffer"), "10" ("string"), "707" ("string"), "06" ("string"), "00" ("string"), w14033) -> (w14047)
            n8822 = String To Byte Array(string=w14047) -> (unsigned byte array=w14052)
            n8823 = for {
              tunnel: w14052 -> [w14081] mode=indexing